vi "HFRR ADV v039.vi"() -> ()   [LabVIEW 2025] (continued)
                    n2649 = local read "Elapsed time"() -> (w3262:dbl)
                    n2650 = local read "AIR TEMP"() -> (w3235:dbl)
                    n2651 = local read "PID-out"() -> (w3240:dbl)
                    n2652 = local write "Temperature ( Deg C )"(w3231) -> ()
                    n2653 = Number To Fractional String(number=w3209, width (-)=i16 9 ("precision (6)"), precision (6)=i16 6) -> (F-format string=w3255:string)  [unwired: 1 in]
                    n2654 = Number To Fractional String(number=w3235, width (-)=i16 9 ("precision (6)"), precision (6)=i16 3) -> (F-format string=w3254:string)  [unwired: 1 in]
                    n2655 = Number To Fractional String(number=w3231, width (-)=i16 9 ("precision (6)"), precision (6)=i16 3) -> (F-format string=w3251:string)  [unwired: 1 in]
                    n2656 = Number To Fractional String(number=w3230, width (-)=i16 9 ("precision (6)"), precision (6)=i16 3) -> (F-format string=w3248:string)  [unwired: 1 in]
                    n2657 = Number To Fractional String(number=0.0, width (-)=i16 9 ("precision (6)"), precision (6)=i16 3) -> (F-format string=w3245:string)  [unwired: 1 in]
                    n2658 = Number To Fractional String(number=w3240, width (-)=i16 9 ("precision (6)"), precision (6)=i16 3) -> (F-format string=w3241:string)  [unwired: 1 in]
                    n2659 = Number To Fractional String(number=w3237, width (-)=i16 9 ("precision (6)"), precision (6)=i16 3) -> (F-format string=w3236:string)  [unwired: 1 in]
                    n2660 = Number To Fractional String(number=w3228, width (-)=i16 9 ("precision (6)"), precision (6)=i16 6) -> (F-format string=w3263:string)  [unwired: 1 in]
                    n2661 = Number To Fractional String(number=w3262, width (-)=i16 14 ("precision (6)"), precision (6)=i16 3) -> (F-format string=w3264:string)  [unwired: 1 in]
                    n2662 = Bundle("y"=1.02, "LVDT STROKE DISPLAY"=w3209, "y"=0.98) -> (w3229:T31)  [unwired: 1 in]
                    n2663 = Number To Fractional String(number="Ambient Humidity :", width (-)=i16 9 ("precision (6)"), precision (6)=i16 6) -> (F-format string=w3221:string)  [unwired: 1 in]
                    n2664 = local read "RUN"() -> (w3227:bool)
                    n2665 = case shown="True" w3227 {
                      tunnel: w3229 -> [_ w3280]
                      tunnel: w3209 -> [_ w3279]
                      tunnel: w3209 -> [_ w3277]
                      tunnel: w3209 -> [_ w3278]
                      frame False {
                      }
                      frame True {
                        "Stroke ( mm )" <- w3280
                        "Stroke ( mm )" <- w3280
                        "Stroke 4" <- w3279
                        "Stroke 3" <- w3277
                        "Stroke 2" <- w3278
                        "measured_stroke" <- w3277
                      }
                    }
                    n2666 = Concatenate Strings(w3264, w3223, w3263, w3223, w3255, w3223, w3254, w3223, w3251, w3223, w3248, w3223, w3245, w3223, w3241, w3223, w3236, w3223, w3221, "\r") -> (w3261:string)
                    n2667 = call <vilib>:"Write Characters To File.vi"("append to file? (new file:F)"=TRUE, "character string"=w3261, "file path (dialog if empty)"=w3214) -> ()  [unwired: 2 in, 1 out]
                    "refresh flag" <- TRUE ("refresh flag")
                    "LVDT STROKE Actual" <- w3207
                  }
                }
                n2668 = case shown="True" w3129 {
                  tunnel: w3139 -> [_ w3165]
                  tunnel: w3144 -> [_ w3175]
                  tunnel: [0.0 w3171] -> _
                  tunnel: w3138 -> [_ w3170]
                  tunnel: [0.0 w3169] -> _
                  tunnel: w3128 -> [_ w3169]
                  tunnel: w3142 -> [w3158 _]
                  frame False {
                    n2669 = local write "acq timer"(w3158) -> ()
                    n2670 = local write "Test Duration Status"(0.0 ("Test Duration Status")) -> ()
                  }
                  frame True {
                    n2671 = local read "Set Hz"() -> (w3172:dbl)
                    n2672 = local write "Elapsed time"(w3165) -> ()
                    n2673 = local read "test time"() -> (w3164:dbl)
                    n2674 = Multiply(x=w3175, y=w3172) -> (x*y=w3174:dbl)
                    n2675 = case shown="False" w3170 {
                      tunnel: w3174 -> [w3176 _]
                      tunnel: [w3176 1.0] -> w3171
                      frame False {
                        n2676 = local write "Cycles elapsed"(w3176) -> ()
                      }
                      frame True {
                      }
                    }
                    n2677 = Greater?(x=w3165, y=w3164) -> (0:w3173:bool)
                    n2678 = Subtract(x=w3164, y=w3165) -> (x-y=w3163:dbl)
                    n2679 = Multiply(x=w3163, y=60.0) -> (x*y=w3162:dbl)
                    n2680 = local write "Time Remaining"(w3162) -> ()
                    n2681 = local write "Remaining Time"(w3162) -> ()
                    n2682 = case shown="True" w3173 {
                      frame False {
                      }
                      frame True {
                        n2683 = stacked-sequence {
                          frame #0 {
                            w3181 = T19."Enabled" ("Disabled")
                            w3180 = FALSE ("TEST FILE NAM,E SAVED")
                            w3182 = "" ("FILE")
                            w3183 = TRUE ("Visible")
                            n2684 = local write "Humidity"(FALSE ("Humidity")) -> ()
                            n2685 = local write "RUN"(FALSE ("OK Button 2")) -> ()
                            n2686 = local write "Heater Button"(FALSE ("Heater Button")) -> ()
                            n2687 = local write "Auto Start Test"(FALSE ("Auto Start Test")) -> ()
                            n2688 = local write "TestCompFlg"(TRUE ("StpFlg")) -> ()
                            n2689 = local read "Humidity ( %RH )"() -> (→"Rh After":dbl)
                            n2690 = property on="STOP 2" class="Bool (strict)"("Disabled"=u8 0) -> ()  [unwired: 2 in, 2 out]
                            n2691 = local read "EVENT LOG"() -> (w3188:string)
                            n2692 = call "Event Log.vi"("Content"="Test Completed", "EVENT LOG"=w3188) -> ("EVENT LOG"=w3187:string)  [unwired: 8 in, 1 out]
                            n2693 = property on="RUN" class="Bool (strict)"("Visible"=w3183) -> ()  [unwired: 2 in, 2 out]
                            n2694 = property on="Auto Start Test" class="Bool (strict)"("Visible"=w3183) -> ()  [unwired: 2 in, 2 out]
                            n2695 = local write "Batch Ref Num :"(w3182) -> ()
                            n2696 = local write "FILE"(w3182) -> ()
                            n2697 = local write "EVENT LOG"(w3187) -> ()
                            n2698 = local write "TEST FILE NAM,E SAVED"(w3180) -> ()
                            n2699 = local write "Fuel Discription :"(w3182) -> ()
                            n2700 = local write "START TEMP"(w3180) -> ()
                            n2701 = local write "Remarks :"(w3182) -> ()
                            n2702 = local write "Main Dashboard Buttons"(T1."Imaging" ("Main Dashboard Buttons")) -> ()
                            n2703 = local write "Main Tab"(T2."Adv Scar" ("Main Tab")) -> ()
                            n2704 = property on="FRICVALZ 2" class="Bool (strict)"("DisabledEnum"=w3181) -> ()  [unwired: 2 in, 2 out]
                            n2705 = property on="FRICVALZ 3" class="Bool (strict)"("DisabledEnum"=w3181) -> ()  [unwired: 2 in, 2 out]
                            n2706 = property on="FRICVALZ 4" class="Bool (strict)"("DisabledEnum"=w3181) -> ()  [unwired: 2 in, 2 out]
                          }
                          frame #1 {
                            n2707 = Wait (ms)(milliseconds to wait=u32 1500) -> ()  [unwired: 1 out]
                          }
                          frame #2 {
                            n2708 = local write "Due Write"("VC;0") -> ()
                          }
                          frame #3 {
                            n2709 = Wait (ms)(milliseconds to wait=u32 1500) -> ()  [unwired: 1 out]
                          }
                          frame #4 {
                            n2710 = local write "Due Write"("VC;0") -> ()
                          }
                          frame #5 {
                            n2711 = Wait (ms)(milliseconds to wait=u32 1500) -> ()  [unwired: 1 out]
                          }
                          frame #6 {
                            n2712 = local write "Due Write"("ST;0") -> ()
                          }
                          frame #7 {
                            n2713 = local write "measured_stroke"(0.0 ("measured_stroke")) -> ()
                            n2714 = Wait (ms)(milliseconds to wait=u32 1500) -> ()  [unwired: 1 out]
                          }
                          frame #8 {
                            n2715 = local write "Due Write"("HE;0") -> ()
                            n2716 = local write "Humidity 2"(TRUE ("Humidity")) -> ()
                          }
                        }
                      }
                    }
                    n2717 = Divide(x=w3165, y=w3164) -> (x/y=w3168:dbl)
                    n2718 = Multiply(x=w3168, y=100.0) -> (x*y=w3166:dbl)
                    n2719 = local write "Test Duration Status"(w3166) -> ()
                  }
                }
              }
              frame #2 {
                n2720 = case shown="True" "Heater Button" {
                  tunnel: [0.0 ("output") w3303] -> w3281
                  frame False {
                    w3284 = TRUE ("tmpchk")
                    n2721 = local read "TEMP"() -> (w3285:dbl)
                    n2722 = local write "Temp ini"(w3285) -> ()
                    n2723 = local write "Reset 4"(w3284) -> ()
                    n2724 = local write "tmpchk"(w3284) -> ()
                    n2725 = local write "reinit"(TRUE ("reinit")) -> ()
                    n2726 = local write "manual temp log"(TRUE ("manual temp log")) -> ()
                  }
                  frame True {
                    # "Logic to turn off\nthe heater when \ntemp is not rising.\nTime - 60 sec\nDelta t- 5°c"
                    n2727 = local read "Temp ini"() -> (w3292:dbl)
                    n2728 = local read "Auto Start Test"() -> (w3288:bool)
                    n2729 = Less?(x=w3292, y=53.0) -> (x < y?=w3290:bool)
                    n2730 = case shown="False" w3288 {
                      frame False {
                        n2731 = local read "Set Temp"() -> (w3312:dbl)
                        n2732 = local read "TEMP"() -> (w3311:dbl)
                        n2733 = Subtract(x=w3312, y=w3311) -> (x-y=w3310:dbl)
                        n2734 = Absolute Value(x=w3310) -> (abs(x)=w3309:dbl)
                        n2735 = Less?(x=w3309, y=0.5) -> (x < y?=w3307:bool)
                        n2736 = case shown="True" w3307 {
                          tunnel: "manual temp log" -> [_ w3313]
                          frame False {
                          }
                          frame True {
                            n2737 = case shown="True" w3313 {
                              selector: w3313 -> [_ w3314]
                              frame False {
                              }
                              frame True {
                                # "#Event log"
                                n2738 = Not(x=w3314) -> (.not. x?=w3315:bool)
                                n2739 = local write "manual temp log"(w3315) -> ()
                                n2740 = local read "EVENT LOG"() -> (w3318:string)
                                n2741 = call "Event Log.vi"("Content"="Target Temperature reached", "EVENT LOG"=w3318) -> ("EVENT LOG"=w3317:string)  [unwired: 8 in, 1 out]
                                n2742 = local write "EVENT LOG"(w3317) -> ()
                              }
                            }
                          }
                        }
                      }
                      frame True {
                        n2743 = local write "manual temp log"(TRUE ("manual temp log")) -> ()
                      }
                    }
                    n2744 = And(x="tmpchk", y=w3290) -> (x .and. y?=w3293:bool)
                    n2745 = case shown="True" w3293 {
                      frame False {
                      }
                      frame True {
                        n2746 = call "Elapsed Time8"("Time Target (s)"=300.0, "Reset"="Reset 4") -> ("Time has Elapsed"=w3320:bool)  [unwired: 10 in, 7 out]
                        n2747 = flat-sequence {
                          tunnel: w3320 -> [_]
                          frame #0 {
                            n2748 = local write "Reset 4"(FALSE ("Reset 4")) -> ()
                          }
                        }
                        n2749 = case shown="True" w3320 {
                          frame False {
                          }
                          frame True {
                            n2750 = local read "Temp ini"() -> (w3327:dbl)
                            n2751 = Add(x=w3327, y=5.0) -> (x+y=w3325:dbl)
                            n2752 = local read "TEMP"() -> (w3328:dbl)
                            n2753 = Greater?(x=w3328, y=w3325) -> (0:w3326:bool)
                            n2754 = case shown="False" w3326 {
                              frame False {
                                n2755 = local write "Heater Button"(FALSE ("Heater Button")) -> ()
                              }
                              frame True {
                                n2756 = local write "tmpchk"(FALSE ("tmpchk")) -> ()
                              }
                            }
                          }
                        }
                      }
                    }
                    n2757 = local read "Set Temp"() -> (w3301:dbl)
                    n2758 = local read "TEMP"() -> (w3295:dbl)
                    n2759 = call-poly <vilib>:"PID.vi"("reinitialize? (F)"="reinit", "dt (s)"=-1.0, "process variable"=w3295, "setpoint"=w3301) -> ("output"=w3298:dbl)  [unwired: 6 in, 1 out]
                    n2760 = Subtract(x=w3301, y=w3295) -> (x-y=w3302:dbl)
                    n2761 = Add(x=w3301, y=0.5) -> (x+y=w3299:dbl)
                    n2762 = Greater Or Equal?(x=w3295, y=w3299) -> ()  [unwired: 1 out]
                    n2763 = Select(t=0.0, s=FALSE, f=w3298) -> (s? t:f=w3297:dbl)
                    "PID output" <- w3297
                    n2764 = flat-sequence {
                      tunnel: w3297 -> [w3331]
                      tunnel: [w3331] -> w3303
                      frame #0 {
                        n2765 = local write "reinit"(FALSE ("reinit")) -> ()
                      }
                    }
                    n2766 = Bundle(w3302, "output"=w3297, "TEMP"=w3295) -> ()  [unwired: 1 in, 1 out]
                  }
                }
                "PID-out" <- w3281
              }
              frame #3 {
                n2767 = local read "TEMP"() -> (w3333:dbl)
                n2768 = Greater Or Equal?(x=w3333, y="Set Temp 2") -> (x >= y?=w3338:bool)
                n2769 = case shown="True" w3338 {
                  tunnel: [FALSE TRUE] -> w3336
                  frame False {
                  }
                  frame True {
                  }
                }
                "Status 13" <- w3336
                n2770 = And(x=w3336, y="trip1 8") -> (x .and. y?=w3335:bool)
                n2771 = case shown="True" w3335 {
                  frame False {
                    n2772 = local write "Heater Trip Temp"(TRUE ("Heater Trip Temp")) -> ()
                  }
                  frame True {
                    w3341 = FALSE ("OK Button 2")
                    n2773 = case shown="True" "Heater Trip Temp" {
                      selector: "Heater Trip Temp" -> [_ w3343]
                      frame False {
                      }
                      frame True {
                        n2774 = Not(x=w3343) -> (.not. x?=w3342:bool)
                        n2775 = local read "EVENT LOG"() -> (w3346:string)
                        n2776 = local write "Heater Trip Temp"(w3342) -> ()
                        n2777 = call "Event Log.vi"("Content"="Heater Trip", "EVENT LOG"=w3346) -> ("EVENT LOG"=w3345:string)  [unwired: 8 in, 1 out]
                        n2778 = local write "EVENT LOG"(w3345) -> ()
                      }
                    }
                    n2779 = local write "RUN"(w3341) -> ()
                    n2780 = property on="Auto Start Test" class="Bool (strict)"("Value"=w3341) -> ()  [unwired: 2 in, 2 out]
                    n2781 = local write "Heater Button"(w3341) -> ()
                  }
                }
              }
            }
            n2782 = case shown="False" w3052 {
              frame False {
                n2783 = disable-structure shown="Disabled" {
                  frame Disabled {
                    n2784 = stacked-sequence {
                      frame #0 {
                        n2785 = local write "RUN"(FALSE ("OK Button 2")) -> ()
                      }
                      frame #1 {
                      }
                    }
                  }
                  frame Enabled {
                  }
                }
              }
              frame True {
              }
            }
          }
        }
        n2786 = local read "Reset Graph"() -> (w2949:bool)
        n2787 = case shown="True" w2949 {
          selector: w2949 -> [_ w2966]
          frame False {
          }
          frame True {
            w2980 = 0.0 ("X Scale.Range:Maximum")
            n2788 = Not(x=w2966) -> (.not. x?=w2965:bool)
            n2789 = local write "Reset Graph"(w2965) -> ()
            n2790 = property on="Electrical Contact Resistance ( % )" class="WFChart (strict)"("XScale.Maximum"=600.0 ("X Scale.Range:Maximum"), "XScale.Minimum"=0.0 ("X Scale.Range:Minimum"), "YScale.Maximum"=100.0 ("Y Scale.Range:Maximum"), "YScale.Minimum"=0.0 ("Y Scale.Range:Minimum")) -> ()  [unwired: 2 in, 2 out]
            n2791 = property on="Frictional Force ( N )" class="WFChart (strict)"("XScale.Maximum"=600.0 ("X Scale.Range:Maximum"), "XScale.Minimum"=0.0 ("X Scale.Range:Minimum"), "YScale.Maximum"=100.0 ("Y Scale.Range:Maximum"), "YScale.Minimum"=0.0 ("Y Scale.Range:Minimum")) -> ()  [unwired: 2 in, 2 out]
            n2792 = property on="Temperature ( Deg C )" class="WFChart (strict)"("XScale.Maximum"=600.0 ("X Scale.Range:Maximum"), "XScale.Minimum"=0.0 ("X Scale.Range:Minimum"), "YScale.Maximum"=100.0 ("Y Scale.Range:Maximum"), "YScale.Minimum"=0.0 ("Y Scale.Range:Minimum")) -> ()  [unwired: 2 in, 2 out]
            n2793 = property on="Stroke ( mm )" class="WFChart (strict)"("XScale.Maximum"=600.0 ("X Scale.Range:Maximum"), "XScale.Minimum"=0.0 ("X Scale.Range:Minimum"), "YScale.Maximum"=100.0 ("Y Scale.Range:Maximum"), "YScale.Minimum"=0.0 ("Y Scale.Range:Minimum")) -> ()  [unwired: 2 in, 2 out]
            n2794 = property on="Coefficient of Friction" class="WFChart (strict)"("XScale.Maximum"=600.0 ("X Scale.Range:Maximum"), "XScale.Minimum"=0.0 ("X Scale.Range:Minimum"), "YScale.Maximum"=100.0 ("Y Scale.Range:Maximum"), "YScale.Minimum"=0.0 ("Y Scale.Range:Minimum")) -> ()  [unwired: 2 in, 2 out]
            n2795 = property on="Electrical Contact Resistance ( % )" class="WFChart (strict)"("XScale.Minimum"=0.0 ("X Scale.Range:Minimum"), "XScale.Maximum"=600.0 ("X Scale.Range:Maximum"), "YScale.Minimum"=0.0 ("Y Scale.Range:Minimum"), "YScale.Maximum"=100.0 ("Y Scale.Range:Maximum")) -> ()  [unwired: 2 in, 2 out]
            n2796 = property on="Temperature ( Deg C )" class="WFChart (strict)"("XScale.Minimum"=0.0 ("X Scale.Range:Minimum"), "XScale.Maximum"=600.0 ("X Scale.Range:Maximum"), "YScale.Minimum"=0.0 ("Y Scale.Range:Minimum"), "YScale.Maximum"=100.0 ("Y Scale.Range:Maximum")) -> ()  [unwired: 2 in, 2 out]
            n2797 = property on="Coefficient of Friction" class="WFChart (strict)"("XScale.Minimum"=0.0 ("X Scale.Range:Minimum"), "XScale.Maximum"=600.0 ("X Scale.Range:Maximum"), "YScale.Maximum"=1.0 ("X Scale.Range:Minimum"), "YScale.Minimum"=0.0 ("X Scale.Range:Minimum")) -> ()  [unwired: 2 in, 2 out]
            n2798 = property on="Frictional Force ( N )" class="WFChart (strict)"("XScale.Maximum"=600.0 ("X Scale.Range:Maximum"), "XScale.Minimum"=w2980, "YScale.Maximum"=10.0 ("Y Scale.Range:Maximum"), "YScale.Minimum"=w2980) -> ()  [unwired: 2 in, 2 out]
            n2799 = property on="Stroke ( mm )" class="WFChart (strict)"("XScale.Maximum"=600.0 ("X Scale.Range:Maximum"), "XScale.Minimum"=0.0 ("X Scale.Range:Minimum"), "YScale.Maximum"=100.0 ("Y Scale.Range:Maximum"), "YScale.Minimum"=0.0 ("Y Scale.Range:Minimum")) -> ()  [unwired: 2 in, 2 out]
          }
        }
      }
      frame "Compare Files" {
        # "Elapsed time\ncof\nstroke\nAir temp\nTemp\nHumidity"
        n2800 = case shown="True" "RSTV1 2" {
          frame False {
          }
          frame True {
            n2801 = property on="Humidity ( %RH )" class="XYGraph (strict)"("Y Scale.Display Format:Precision"=u8 0 ("Y Scale.Format & Precision:Precision")) -> ()  [unwired: 2 in, 2 out]
            n2802 = property on="Humidity ( %RH )" class="XYGraph (strict)"("X Scale.Range:Minimum"=0.0, "X Scale.Range:Maximum"=75.0, "Y Scale.Range:Minimum"=48.0, "Y Scale.Range:Maximum"=58.0) -> ()  [unwired: 2 in, 2 out]
          }
        }
        n2803 = case shown="True" "RST CP 2" {
          frame False {
          }
          frame True {
            n2804 = property on="XY Graph 13" class="XYGraph (strict)"("Y Scale.Display Format:Precision"=u8 0 ("Y Scale.Format & Precision:Precision")) -> ()  [unwired: 2 in, 2 out]
            n2805 = property on="XY Graph 13" class="XYGraph (strict)"("X Scale.Range:Minimum"=0.0, "X Scale.Range:Maximum"=75.0, "Y Scale.Range:Minimum"=0.0, "Y Scale.Range:Maximum"=100.0) -> ()  [unwired: 2 in, 2 out]
          }
        }
        n2806 = case shown="True" "RST CP" {
          frame False {
          }
          frame True {
            n2807 = property on="Sample Temperature ( °C )" class="XYGraph (strict)"("Y Scale.Display Format:Precision"=u8 2 ("Y Scale.Format & Precision:Precision")) -> ()  [unwired: 2 in, 2 out]
            n2808 = property on="Sample Temperature ( °C )" class="XYGraph (strict)"("X Scale.Range:Minimum"=0.0, "X Scale.Range:Maximum"=75.0, "Y Scale.Range:Minimum"=58.0, "Y Scale.Range:Maximum"=62.0) -> ()  [unwired: 2 in, 2 out]
          }
        }
        n2809 = case shown="True" "RSTV1 3" {
          frame False {
          }
          frame True {
            n2810 = property on="Air Temperature  ( °C )" class="XYGraph (strict)"("Y Scale.Display Format:Precision"=u8 2 ("Y Scale.Format & Precision:Precision")) -> ()  [unwired: 2 in, 2 out]
            n2811 = property on="Air Temperature  ( °C )" class="XYGraph (strict)"("X Scale.Range:Minimum"=0.0 ("Y Scale.Range:Minimum"), "X Scale.Range:Maximum"=75.0 ("Y Scale.Range:Maximum"), "Y Scale.Range:Minimum"=20.0 ("X Scale.Range:Minimum"), "Y Scale.Range:Maximum"=26.0 ("X Scale.Range:Maximum")) -> ()  [unwired: 2 in, 2 out]
          }
        }
        n2812 = case shown="True" "RSTV1 4" {
          frame False {
          }
          frame True {
            n2813 = property on="Stroke ( mm )" class="XYGraph (strict)"("Y Scale.Display Format:Precision"=u8 2 ("Y Scale.Format & Precision:Precision")) -> ()  [unwired: 2 in, 2 out]
            n2814 = property on="Stroke ( mm )" class="XYGraph (strict)"("X Scale.Range:Minimum"=0.0 ("Y Scale.Range:Maximum"), "X Scale.Range:Maximum"=75.0 ("X Scale.Range:Minimum"), "Y Scale.Range:Minimum"=0.98, "Y Scale.Range:Maximum"=1.02) -> ()  [unwired: 2 in, 2 out]
          }
        }
        n2815 = case shown="True" "rstv2" {
          frame False {
          }
          frame True {
            n2816 = property on="Coefficient Of Friction" class="XYGraph (strict)"("Y Scale.Display Format:Precision"=u8 3 ("Y Scale.Format & Precision:Precision")) -> ()  [unwired: 2 in, 2 out]
            n2817 = property on="Coefficient Of Friction" class="XYGraph (strict)"("X Scale.Range:Minimum"=0.0 ("Y Scale.Range:Maximum"), "X Scale.Range:Maximum"=75.0, "Y Scale.Range:Minimum"=0.0, "Y Scale.Range:Maximum"=1.0 ("X Scale.Range:Minimum")) -> ()  [unwired: 2 in, 2 out]
          }
        }
        n2818 = case shown="True" "RST CP 3" {
          frame False {
          }
          frame True {
            n2819 = property on="Air Temp ( °C ) vs Humidity ( % RH )" class="XYGraph (strict)"("X Scale.Range:Minimum"=18.0, "X Scale.Range:Maximum"=28.0 ("X Scale.Range:Minimum"), "Y Scale.Range:Minimum"=30.0 ("X Scale.Range:Minimum"), "Y Scale.Range:Maximum"=70.0 ("X Scale.Range:Minimum")) -> ()  [unwired: 2 in, 2 out]
          }
        }
        n2820 = case shown="True" "OPEN 1" {
          frame False {
          }
          frame True {
            (unwired) 0  # existing file
            w3622 = "Choose a datalog file to open"  # prompt
            n2821 = local write "OPEN 1"(FALSE ("OPEN 1")) -> ()
            n2822 = String To Path(string="C:\\LAB-IQ\\Data\\") -> (path=w3607:path)
            n2823 = File Dialog(6:"*.dgf" ("pattern"), 7:w3622, 11:w3607) -> (0:w3605:errorcluster, 3:w3613:path)  [unwired: 4 in, 2 out]
            n2824 = Unbundle(w3605) -> ()  [unwired: 3 out]
            n2825 = Strip Path(path=w3613) -> (name=w3612:string)  [unwired: 1 out]
            n2826 = Path To String(path=w3613) -> (string=w3608:string)
            "string1" <- w3608
            n2827 = Match Pattern(string=w3612, regular expression=".dgf") -> (before substring=→"String Control":string)  [unwired: 1 in, 3 out]
            n2828 = Match Pattern(string=w3608, regular expression=".dgf" ("substring (\"\")")) -> (before substring=w3618:string)  [unwired: 1 in, 3 out]
            n2829 = Concatenate Strings(w3618, ".duf" ("Substring")) -> (w3614:string)
            n2830 = String To Path(string=w3614) -> (path=w3619:path)
            n2831 = call <vilib>:"Read Characters From File.vi"("file path (dialog if empty)"=w3619, "start of read offset (chars.:0)"=60 ("start of read offset (chars.: 0)")) -> ("character string"=→"String Control 2":string)  [unwired: 4 in, 3 out]
          }
        }
        n2832 = case shown="True" "OPEN 2" {
          frame False {
          }
          frame True {
            (unwired) 0  # existing file
            w3640 = "Choose a datalog file to open"  # prompt
            n2833 = local write "OPEN 2"(FALSE ("OPEN 1")) -> ()
            n2834 = String To Path(string="C:\\LAB-IQ\\Data\\") -> (path=w3625:path)
            n2835 = File Dialog(6:"*.dgf" ("pattern"), 7:w3640, 11:w3625) -> (0:w3623:errorcluster, 3:w3631:path)  [unwired: 4 in, 2 out]
            n2836 = Unbundle(w3623) -> ()  [unwired: 3 out]
            n2837 = Strip Path(path=w3631) -> (name=w3629:string)  [unwired: 1 out]
            n2838 = Path To String(path=w3631) -> (string=w3626:string)
            "string1 2" <- w3626
            n2839 = Match Pattern(string=w3629, regular expression=".dgf") -> (before substring=→"String Control 3":string)  [unwired: 1 in, 3 out]
            n2840 = Match Pattern(string=w3626, regular expression=".dgf" ("substring (\"\")")) -> (before substring=w3637:string)  [unwired: 1 in, 3 out]
            n2841 = Concatenate Strings(w3637, ".duf" ("Substring")) -> (w3634:string)
            n2842 = String To Path(string=w3634) -> (path=w3632:path)
            n2843 = call <vilib>:"Read Characters From File.vi"("file path (dialog if empty)"=w3632, "start of read offset (chars.:0)"=60 ("start of read offset (chars.: 0)")) -> ("character string"=→"String Control 4":string)  [unwired: 4 in, 3 out]
          }
        }
        n2844 = case shown="True" "OPEN 3" {
          frame False {
          }
          frame True {
            (unwired) 0  # existing file
            w3658 = "Choose a datalog file to open"  # prompt
            n2845 = local write "OPEN 3"(FALSE ("OPEN 1")) -> ()
            n2846 = String To Path(string="C:\\LAB-IQ\\Data\\") -> (path=w3643:path)
            n2847 = File Dialog(6:"*.dgf" ("pattern"), 7:w3658, 11:w3643) -> (0:w3641:errorcluster, 3:w3649:path)  [unwired: 4 in, 2 out]
            n2848 = Unbundle(w3641) -> ()  [unwired: 3 out]
            n2849 = Strip Path(path=w3649) -> (name=w3647:string)  [unwired: 1 out]
            n2850 = Path To String(path=w3649) -> (string=w3644:string)
            "string1 3" <- w3644
            n2851 = Match Pattern(string=w3647, regular expression=".dgf") -> (before substring=→"String Control 5":string)  [unwired: 1 in, 3 out]
            n2852 = Match Pattern(string=w3644, regular expression=".dgf" ("substring (\"\")")) -> (before substring=w3654:string)  [unwired: 1 in, 3 out]
            n2853 = Concatenate Strings(w3654, ".duf" ("Substring")) -> (w3651:string)
            n2854 = String To Path(string=w3651) -> (path=w3655:path)
            n2855 = call <vilib>:"Read Characters From File.vi"("file path (dialog if empty)"=w3655, "start of read offset (chars.:0)"=60 ("start of read offset (chars.: 0)")) -> ("character string"=→"String Control 6":string)  [unwired: 4 in, 3 out]
          }
        }
        n2856 = case shown="True" "OPEN 4" {
          frame False {
          }
          frame True {
            (unwired) 0  # existing file
            w3676 = "Choose a datalog file to open"  # prompt
            n2857 = local write "OPEN 4"(FALSE ("OPEN 1")) -> ()
            n2858 = String To Path(string="C:\\LAB-IQ\\Data\\") -> (path=w3661:path)
            n2859 = File Dialog(6:"*.dgf" ("pattern"), 7:w3676, 11:w3661) -> (0:w3659:errorcluster, 3:w3667:path)  [unwired: 4 in, 2 out]
            n2860 = Unbundle(w3659) -> ()  [unwired: 3 out]
            n2861 = Strip Path(path=w3667) -> (name=w3665:string)  [unwired: 1 out]
            n2862 = Path To String(path=w3667) -> (string=w3662:string)
            "string1 4" <- w3662
            n2863 = Match Pattern(string=w3665, regular expression=".dgf") -> (before substring=→"String Control 7":string)  [unwired: 1 in, 3 out]
            n2864 = Match Pattern(string=w3662, regular expression=".dgf" ("substring (\"\")")) -> (before substring=w3672:string)  [unwired: 1 in, 3 out]
            n2865 = Concatenate Strings(w3672, ".duf" ("Substring")) -> (w3669:string)
            n2866 = String To Path(string=w3669) -> (path=w3673:path)
            n2867 = call <vilib>:"Read Characters From File.vi"("file path (dialog if empty)"=w3673, "start of read offset (chars.:0)"=60 ("start of read offset (chars.: 0)")) -> ("character string"=→"String Control 8":string)  [unwired: 4 in, 3 out]
          }
        }
      }
      frame "About" {
        # "Elapsed time\ncof\nstroke\nmean pos\nTemp\nHumidity"
        n2868 = disable-structure shown="Disabled" {
          frame Disabled {
            n2869 = case shown="True" "Export" {
              frame False {
              }
              frame True {
                w3698 = "                                      " ("string")
                w3700 = "\r"
                (unwired) i16 6 ("width (-)")
                w3777 = "\r"
                w3709 = "\r"
                n2870 = local write "Export"(FALSE ("Export")) -> ()
                n2871 = local read "String 29"() -> (w3746:string)
                n2872 = local read "String 34"() -> (w3734:string)
                n2873 = local read "String 35"() -> (w3729:string)
                n2874 = local read "String 37"() -> (w3725:string)
                n2875 = local read "String 36"() -> (w3722:string)
                n2876 = local read "String 38"() -> (w3719:string)
                n2877 = local read "String 39"() -> (w3716:string)
                n2878 = Match Pattern(string=w3746, regular expression=".dwm") -> (before substring=w3742:string)  [unwired: 1 in, 3 out]
                "before substring" <- w3742
                n2879 = local read "S 38"() -> (w3737:string)
                n2880 = local read "S 39"() -> (w3730:string)
                n2881 = local read "Temperature before test 2"() -> (w3766:dbl)
                n2882 = local read "Temperature after test 2"() -> (w3771:dbl)
                n2883 = local read "Humidity before test 2"() -> (w3752:dbl)
                n2884 = local read "Humidity after test 2"() -> (w3767:dbl)
                n2885 = local read "MWSD 2"() -> (w3763:dbl)
                n2886 = local read "WS1.4 2"() -> (w3779:dbl)
                n2887 = local read "HCF 2"() -> (w3775:dbl)
                n2888 = local read "AVP 2"() -> (w3764:dbl)
                n2889 = Concatenate Strings("1," ("string"), w3737) -> (w3736:string)
                n2890 = Concatenate Strings("2," ("string"), w3734) -> (w3733:string)
                n2891 = Concatenate Strings("3," ("string"), w3730) -> (w3732:string)
                n2892 = Concatenate Strings("4," ("string"), w3729) -> (w3728:string)
                n2893 = Concatenate Strings("5," ("string"), w3725) -> (w3726:string)
                n2894 = Concatenate Strings("6," ("string"), w3722) -> (w3723:string)
                n2895 = Concatenate Strings("7," ("string"), w3719) -> (w3720:string)
                n2896 = Concatenate Strings("8," ("string"), w3716) -> (w3717:string)
                n2897 = local read "Sample ID"() -> (w3784:string)
                n2898 = case shown="\"xlx\"" "Select File Type" {
                  tunnel: w3742 -> [w3787 w3789 w3791]
                  tunnel: [w3785 w3790 w3792] -> w3741
                  frame "xlx" {
                    n2899 = Concatenate Strings(w3787, ".xls" ("string")) -> (w3785:string)
                  }
                  frame "csv" {
                    n2900 = Concatenate Strings(w3789, ".csv" ("string")) -> (w3790:string)
                  }
                  frame "txt" {
                    n2901 = Concatenate Strings(w3791, ".txt" ("string")) -> (w3792:string)
                  }
                }
                n2902 = local read "Test Date"() -> (w3783:string)
                n2903 = local read "String 45"() -> (w3697:string)
                n2904 = local read "String 31"() -> (w3782:string)
                n2905 = local read "String 32"() -> (w3781:string)
                n2906 = local read "TITTLE"() -> (w3705:string)
                n2907 = Number To Fractional String(number=w3752, width (-)=i16 6, precision (6)=i16 2) -> (F-format string=w3751:string)  [unwired: 1 in]
                n2908 = Number To Fractional String(number=w3766, width (-)=i16 6, precision (6)=i16 2) -> (F-format string=w3772:string)  [unwired: 1 in]
                n2909 = Number To Fractional String(number=w3767, width (-)=i16 6, precision (6)=i16 2) -> (F-format string=w3765:string)  [unwired: 1 in]
                n2910 = Number To Fractional String(number=w3771, width (-)=i16 6, precision (6)=i16 2) -> (F-format string=w3770:string)  [unwired: 1 in]
                n2911 = Number To Fractional String(number=w3763, width (-)=i16 6, precision (6)=i16 2) -> (F-format string=w3761:string)  [unwired: 1 in]
                n2912 = Number To Fractional String(number=w3764, width (-)=i16 6, precision (6)=i16 2) -> (F-format string=w3762:string)  [unwired: 1 in]
                n2913 = Number To Fractional String(number=w3775, width (-)=i16 6, precision (6)=i16 2) -> (F-format string=w3776:string)  [unwired: 1 in]
                n2914 = Number To Fractional String(number=w3779, precision (6)=i16 2) -> (F-format string=w3780:string)  [unwired: 2 in]
                n2915 = local read "s.NO"() -> (w3699:string)
                n2916 = Concatenate Strings("=" ("string"), w3705) -> (w3704:string)
                n2917 = Concatenate Strings("S.No," ("string"), "                                       Parameters" ("string")) -> (w3710:string)
                n2918 = Concatenate Strings(w3777, w3736, w3751, w3777, w3733, w3772, w3777, w3732, w3765, w3777, w3728, w3770, w3777, w3726, w3761, w3777, w3723, w3762, w3777, w3720, w3776, w3777, w3717, w3780) -> (w3739:string)
                n2919 = Concatenate Strings(w3709, "," ("string"), w3697, w3699, w3698, w3781, w3784, w3698, w3782, w3783, w3709) -> (w3707:string)
                n2920 = local read "Tested by"() -> (w3713:string)
                n2921 = local read "String 33"() -> (w3714:string)
                n2922 = Concatenate Strings("," ("string"), "                                                                             " ("string")) -> (w3702:string)
                n2923 = Concatenate Strings(w3704, w3700, w3707, w3700, w3710, w3739, w3700, w3702, w3714, w3713) -> (→"export":string)
                n2924 = String To Path(string=w3741) -> (path=w3748:path)
                n2925 = local read "export"() -> (w3743:string)
                n2926 = call <vilib>:"Write Characters To File.vi"("append to file? (new file:F)"=FALSE, "character string"=w3743, "file path (dialog if empty)"=w3748) -> ()  [unwired: 2 in, 1 out]
              }
            }
          }
          frame Enabled {
          }
        }
        n2927 = case shown="True" "OK Button 17" {
          frame False {
          }
          frame True {
            (unwired) 0  # existing file
            w4001 = "Choose a datalog file to open"  # prompt
            n2928 = local write "OK Button 17"(FALSE ("OK Button 17")) -> ()
            n2929 = local read "String"() -> (w3996:string)
            n2930 = String To Path(string=w3996) -> (path=w3997:path)
            n2931 = File Dialog(6:"*.duf" ("pattern"), 7:w4001, 11:w3997) -> (0:w3988:errorcluster, 3:w4007:path)  [unwired: 4 in, 2 out]
            n2932 = Unbundle(w3988) -> ()  [unwired: 3 out]
            n2933 = Open/Create/Replace File "Open File"(file path (use dialog)=w4007) -> (refnum out=w3999:refnum<file>)  [unwired: 5 in, 2 out]
            n2934 = Strip Path(path=w4007) -> (name=w4005:string)  [unwired: 1 out]
            n2935 = Path To String(path=w4007) -> (string=w3990:string)
            n2936 = while {
              tunnel: w3999 -> [w4011]
              i -> [w4008]
              stop <- w4009 continue-if-true
              (unwired) TRUE ("line mode (F)")
              n2937 = Read from Text File "Read File"(file (use dialog)=w4011) -> (text=w4010:string)  [unwired: 3 in, 3 out]
              n2938 = local write "Numeric 16"(w4008) -> ()
              n2939 = String Length(string=w4010) -> (length=w4013:i32)
              n2940 = Greater?(x=w4013, y=1) -> (0:w4009:bool)
            }
            n2941 = local write "String 29"(w3990) -> ()
            n2942 = Search and Replace String(input string=w3990, search string=".duf", replace string=".dgf" ("replace string (\"\")")) -> (result string=→"String Indicator 4":string)  [unwired: 5 in, 3 out]
            n2943 = Match Pattern(string=w4005, regular expression=".dwm") -> (before substring=w3989:string)  [unwired: 1 in, 3 out]
            "String Indicator" <- w3989
            n2944 = Match Pattern(string=w3990, regular expression=".dwm" ("substring (\"\")")) -> (before substring=w3991:string)  [unwired: 1 in, 3 out]
            "String Indicator 3" <- w3991
            n2945 = local write "TITTLE 2"(w3989) -> ()
            n2946 = String To Path(string=w3991) -> (path=w3998:path)
            "path" <- w3998
            n2947 = call <vilib>:"Read Characters From File.vi"("file path (dialog if empty)"=w3998, "start of read offset (chars.:0)"=60 ("start of read offset (chars.: 0)")) -> ("character string"=→"String Indicator 2":string)  [unwired: 4 in, 3 out]
          }
        }
        n2948 = call <vilib>:"Query Available Printers.vi"() -> ("system configured printers"=w3690:string[])  [unwired: 9 in, 2 out]
        "System Configured Printers 2" <- w3690
        n2949 = local read "OK Button 16"() -> (w3687:bool)
        n2950 = case shown="True" "OK Button 16" {
          frame False {
          }
          frame True {
            n2951 = stacked-sequence {
              frame #0 {
                n2952 = local read "Numeric 16"() -> (w4015:i32)
                n2953 = local write "Numeric 10"(w4015) -> ()
              }
              frame #1 {
                n2954 = local read "String 29"() -> (w4018:string)
                n2955 = String To Path(string=w4018) -> (path=w4017:path)
                n2956 = Open/Create/Replace File "Open File"(file path (use dialog)=w4017) -> (refnum out=w4019:refnum<file>)  [unwired: 5 in, 2 out]
                n2957 = for {
                  N: 16 -> [_]
                  tunnel: w4019 -> [w4026]
                  i -> [w4022]
                  (unwired) TRUE ("line mode (F)")
                  n2958 = Read from Text File "Read File"(file (use dialog)=w4026) -> (text=w4020:string)  [unwired: 3 in, 3 out]
                  n2959 = Match Pattern(string=w4020, regular expression="(") -> (after substring=w4025:string)  [unwired: 1 in, 3 out]
                  n2960 = Match Pattern(string=w4025, regular expression=")") -> (before substring=w4021:string)  [unwired: 1 in, 3 out]
                  n2961 = case shown="1" w4022 {
                    tunnel: w4021 -> [w4027 w4028 _ _ w4029 w4030 w4031 w4033 w4035 w4037 w4039 w4041 w4043 w4045 _]
                    tunnel: w4020 -> [_ _ _ _ _ _ _ _ _ _ _ _ _ _ _]
                    frame 0 {
                      "TITTLE" <- w4027
                    }
                    frame 1 {
                      "Sample ID" <- w4028
                    }
                    frame 2 {
                    }
                    frame 3 {
                    }
                    frame 4 {
                      "Test Date" <- w4029
                    }
                    frame 5 {
                      "Tested by" <- w4030
                    }
                    frame 6 {
                      n2962 = Fract/Exp String To Number(string=w4031) -> (number=→"Humidity before test 2":dbl)  [unwired: 3 in, 1 out]
                    }
                    frame 7 {
                      n2963 = Fract/Exp String To Number(string=w4033) -> (number=→"Temperature before test 2":dbl)  [unwired: 3 in, 1 out]
                    }
                    frame 8 {
                      n2964 = Fract/Exp String To Number(string=w4035) -> (number=→"Humidity after test 2":dbl)  [unwired: 3 in, 1 out]
                    }
                    frame 9 {
                      n2965 = Fract/Exp String To Number(string=w4037) -> (number=→"Temperature after test 2":dbl)  [unwired: 3 in, 1 out]
                    }
                    frame 10 {
                      n2966 = Fract/Exp String To Number(string=w4039) -> (number=→"MWSD 2":dbl)  [unwired: 3 in, 1 out]
                    }
                    frame 11 {
                      n2967 = Fract/Exp String To Number(string=w4041) -> (number=→"AVP 2":dbl)  [unwired: 3 in, 1 out]
                    }
                    frame 12 {
                      n2968 = Fract/Exp String To Number(string=w4043) -> (number=→"HCF 2":dbl)  [unwired: 3 in, 1 out]
                    }
                    frame 13 {
                      n2969 = Fract/Exp String To Number(string=w4045) -> (number=→"WS1.4 2":dbl)  [unwired: 3 in, 1 out]
                    }
                    frame 14, Default {
                    }
                  }
                }
              }
              frame #2 {
              }
            }
            n2970 = local write "OK Button 16"(FALSE ("OK Button 13")) -> ()
          }
        }
        n2971 = Index Array(array=w3690, index="Select Printer 3") -> (element=w3692:string)
        "Selected Printer" <- w3692
        n2972 = case shown="True" w3687 {
          frame False {
          }
          frame True {
            n2973 = flat-sequence {
              frame #0 {
              }
              frame #1 {
                n2974 = Wait (ms)(milliseconds to wait=u32 100) -> ()  [unwired: 1 out]
              }
              frame #2 {
                n2975 = local write "OK Button 16"(FALSE ("Print 3")) -> ()
              }
            }
          }
        }
        n2976 = case shown="True" "Print" {
          tunnel: w3692 -> [_ w3984]
          frame False {
          }
          frame True {
            (unwired) i16 6 ("width (-)")
            (unwired) "TESTED BY : "
            (unwired) "TESTED DATE :"
            (unwired) "SAMPLE ID : "
            (unwired) "SAMPLE DESIGN : "
            w3942 = "\r"
            w3959 = "\r"
            # "add image"
            n2977 = local read "Sample ID"() -> (w3932:string)
            n2978 = local read "Tested by"() -> (w3935:string)
            n2979 = local read "String 34"() -> (w3922:string)
            n2980 = local read "String 45"() -> (w3902:string)
            n2981 = local read "String 35"() -> (w3917:string)
            n2982 = local read "String 37"() -> (w3915:string)
            n2983 = local read "String 32"() -> (w3937:string)
            n2984 = local read "String 36"() -> (w3912:string)
            n2985 = local read "String 31"() -> (w3936:string)
            n2986 = local read "Test Date"() -> (w3933:string)
            n2987 = local read "String 33"() -> (w3938:string)
            n2988 = local read "String 38"() -> (w3908:string)
            n2989 = local read "String 39"() -> (w3905:string)
            n2990 = local write "Print"(FALSE ("Print FF")) -> ()
            n2991 = local read "S 39"() -> (w3920:string)
            n2992 = local read "S 38"() -> (w3927:string)
            n2993 = local read "Temperature before test 2"() -> (w3958:dbl)
            n2994 = local read "Temperature after test 2"() -> (w3948:dbl)
            n2995 = local read "Humidity before test 2"() -> (w3973:dbl)
            n2996 = local read "Humidity after test 2"() -> (w3957:dbl)
            n2997 = local read "MWSD 2"() -> (w3962:dbl)
            n2998 = local read "WS1.4 2"() -> (w3940:dbl)
            n2999 = Concatenate Strings("2)" ("string"), w3922) -> (w3923:string)
            n3000 = Concatenate Strings("3)" ("string"), w3920) -> (w3921:string)
            n3001 = Concatenate Strings("1)" ("string"), w3927) -> (w3926:string)
            n3002 = Concatenate Strings("4)" ("string"), w3917) -> (w3918:string)
            n3003 = Concatenate Strings("5)" ("string"), w3915) -> (w3914:string)
            n3004 = Concatenate Strings("6)" ("string"), w3912) -> (w3911:string)
            n3005 = Concatenate Strings("7)" ("string"), w3908) -> (w3909:string)
            n3006 = Concatenate Strings("8)" ("string"), w3905) -> (w3906:string)
            n3007 = local read "HCF 2"() -> (w3944:dbl)
            n3008 = local read "AVP 2"() -> (w3961:dbl)
            n3009 = local read "s.NO"() -> (w3903:string)
            n3010 = call <vilib>:"New Report.vi"("report type"=enum16{"Standard Report", "HTML"}."Standard Report") -> ("report out"=w3982:refnum<class "NI_report.lvclass">, "error out"=w3981:errorcluster)  [unwired: 13 in]
            n3011 = local read "TITTLE"() -> (w3934:string)
            n3012 = Concatenate Strings(w3959, w3902, w3903, w3959, w3937, w3932, w3959, w3936, w3933, w3959, w3938, w3935, w3959) -> (w3952:string)
            "test by" <- w3952
            n3013 = Number To Fractional String(number=w3958, width (-)=i16 6, precision (6)=i16 2) -> (F-format string=w3947:string)  [unwired: 1 in]
            n3014 = Number To Fractional String(number=w3957, width (-)=i16 6, precision (6)=i16 2) -> (F-format string=w3960:string)  [unwired: 1 in]
            n3015 = Number To Fractional String(number=w3973, width (-)=i16 6, precision (6)=i16 2) -> (F-format string=w3978:string)  [unwired: 1 in]
            n3016 = Number To Fractional String(number=w3962, width (-)=i16 6, precision (6)=i16 2) -> (F-format string=w3964:string)  [unwired: 1 in]
            n3017 = Number To Fractional String(number=w3948, width (-)=i16 6, precision (6)=i16 2) -> (F-format string=w3949:string)  [unwired: 1 in]
            n3018 = Number To Fractional String(number=w3961, width (-)=i16 6, precision (6)=i16 2) -> (F-format string=w3963:string)  [unwired: 1 in]
            n3019 = Number To Fractional String(number=w3944, width (-)=i16 6, precision (6)=i16 2) -> (F-format string=w3943:string)  [unwired: 1 in]
            n3020 = Number To Fractional String(number=w3940, precision (6)=i16 2) -> (F-format string=w3939:string)  [unwired: 2 in]
            n3021 = call-dynamic "Set Report Header Text.vi"("report in"=w3982, "center header text"=w3934, "error in (no error)"=w3981) -> ("report out"=w3953:refnum<class "NI_report.lvclass">, "error out"=w3954:errorcluster)  [unwired: 11 in]
            n3022 = Concatenate Strings(w3942, w3926, w3978, w3942, w3923, w3947, w3942, w3921, w3960, w3942, w3918, w3949, w3942, w3914, w3964, w3942, w3911, w3963, w3942, w3909, w3943, w3942, w3906, w3939) -> (w3930:string)
            "export 2" <- w3930
            n3023 = call-poly <vilib>:"Append Report Text.vi"("report in"=w3953, "text"=w3952, "error in (no error)"=w3954) -> ("report out"=w3956:refnum<class "NI_report.lvclass">, "error out"=w3955:errorcluster)  [unwired: 9 in, 2 out]
            n3024 = local read "test by"() -> (w3929:string)
            n3025 = local read "TITTLE"() -> (w3931:string)
            n3026 = call-poly <vilib>:"Append Report Text.vi"("report in"=w3956, "error in (no error)"=w3955) -> ("report out"=w3977:refnum<class "NI_report.lvclass">, "error out"=w3975:errorcluster)  [unwired: 10 in, 2 out]
            n3027 = Concatenate Strings(w3931, w3930, w3929) -> (→"output":string)
            n3028 = call-poly <vilib>:"Append Report Text.vi"("report in"=w3977, "text"=w3930, "error in (no error)"=w3975) -> ("report out"=w3976:refnum<class "NI_report.lvclass">, "error out"=w3974:errorcluster)  [unwired: 9 in, 2 out]
            n3029 = call-dynamic "Print Report.vi"("report in"=w3976, "printer name (default)"=w3984, "error in (no error)"=w3974) -> ("report out"=w3986:refnum<class "NI_report.lvclass">, "error out"=w3987:errorcluster)  [unwired: 11 in]
            n3030 = call-dynamic "Dispose Report.vi"("report in"=w3986, "error in (no error)"=w3987) -> ()  [unwired: 13 in, 1 out]
          }
        }
        n3031 = case shown="True" "Print 2" {
          frame False {
          }
          frame True {
            n3032 = flat-sequence {
              frame #0 {
                n3033 = local read "s.NO"() -> (→"s.NO 2":string)
                n3034 = Wait (ms)(milliseconds to wait=u32 20) -> ()  [unwired: 1 out]
                n3035 = local read "Sample ID  3"() -> (→"Sample ID  6":string)
                n3036 = local read "Sample ID  4"() -> (→"Sample ID  7":string)
                n3037 = local read "Sample ID"() -> (→"Sample ID  2":string)
                n3038 = local read "Tested by"() -> (→"Tested by 2":string)
                n3039 = local read "Test Date"() -> (→"Test Date 2":string)
                n3040 = local read "Humidity after test 3"() -> (→"Humidity after test 4":dbl)
                n3041 = local read "Ref A Test Date :"() -> (→"TITTLE 4":string)
                n3042 = local read "Temperature before test 3"() -> (w3809:dbl)
                n3043 = local read "Temperature before test 3"() -> (→"Temperature after test 5":dbl)
                n3044 = local read "Temperature after test 3"() -> (→"Temperature after test 4":dbl)
                n3045 = local read "Humidity before test 3"() -> (→"Humidity before test 4":dbl)
                n3046 = local write "Temperature before test 3"(w3809) -> ()
                n3047 = local read "image data"() -> (w3800:T16)
                n3048 = String To Path(string="C:\\LAB-IQ\\im\\Temp_resized.jpg") -> (path=w3801:path)
                "path 2" <- w3801
                n3049 = call <vilib>:"Write JPEG File.vi"("image data"=w3800, "path to JPEG file"=w3801) -> ()  [unwired: 8 in, 2 out]
                "Ref A Test Date :" <- "Ref A Test Date :"
                "Ref B Test Date :" <- "Ref B Test Date :"
                "Ref B Scar Value :" <- "Ref B Scar Value :"
                "Ref A Scar Value :" <- "Ref A Scar Value :"
              }
              frame #1 {
                (unwired) HTML_Report_Image_Alignment."MIDDLE" ("alignment (default)")
                w3837 = u16 0 items=["portrait", "landscape"] ("orientation (portrait)")
                (unwired) HTML_Report_Image_Alignment."ABSMIDDLE" ("alignment (default)")
                (unwired) "TESTED BY : "
                (unwired) "TESTED DATE :"
                (unwired) "SAMPLE ID : "
                (unwired) "SAMPLE DESIGN : "
                w3870 = "\r"
                # "add image"
                n3050 = Wait (ms)(milliseconds to wait=u32 20) -> ()  [unwired: 1 out]
                n3051 = local read "Sample ID  2"() -> (w3863:string)
                n3052 = local read "Wear Scar X"() -> (w3835:dbl)
                "Length ( microns ) 2" <- w3835
                n3053 = local read "Wear Scar Y"() -> (w3834:dbl)
                "Wear Scar Y ( microns ) :" <- w3834
                n3054 = local read "Test Date 2"() -> (w3864:string)
                n3055 = local read "Tested by 2"() -> (w3865:string)
                n3056 = local read "String 46"() -> (w3861:string)
                n3057 = local read "String 48"() -> (w3867:string)
                n3058 = local read "String 47"() -> (w3866:string)
                n3059 = local read "String 49"() -> (w3868:string)
                n3060 = local read "String 10"() -> (w3821:string)
                n3061 = local read "s.NO 2"() -> (w3862:string)
                n3062 = Add(x=w3835, y=w3834) -> (x+y=w3833:dbl)
                n3063 = call <vilib>:"New Report.vi"("report type"=enum16{"Standard Report", "HTML"}."HTML") -> ("report out"=w3841:refnum<class "NI_report.lvclass">, "error out"=w3839:errorcluster)  [unwired: 13 in]
                n3064 = Concatenate Strings(w3870, w3861, w3862, w3870, w3867, w3863, w3870, w3866, w3864, w3870, w3868, w3865, w3870) -> (→"test by 2":string)
                n3065 = Concatenate Strings("C:\\LAB-IQ\\Data\\" ("string"), w3821, ".jpg" ("string")) -> ()  [unwired: 1 out]
                n3066 = Divide(x=w3833, y=2.0) -> (x/y=→"Mean Wear ( microns) :":dbl)
                n3067 = call-dynamic "Set Report Orientation.vi"("report in"=w3841, "orientation (portrait)"=w3837, "error in (no error)"=w3839) -> ("report out"=w3840:refnum<class "NI_report.lvclass">, "error out"=w3838:errorcluster)  [unwired: 11 in]
                n3068 = for {
                  N: 5 -> [_]
                  tunnel: w3840 -> [w3891]
                  tunnel: [w3890] -> w3819
                  tunnel: w3838 -> [w3889]
                  tunnel: [w3888] -> w3818
                  n3069 = call-dynamic "Set Report Tab Width.vi"("report in"=w3891, "error in (no error)"=w3889) -> ("report out"=w3890:refnum<class "NI_report.lvclass">, "error out"=w3888:errorcluster)  [unwired: 12 in]
                }
                n3070 = local read "TITTLE"() -> (w3836:string)
                n3071 = call-dynamic "Set Report Header Text.vi"("report in"=w3819, "center header text"=w3836, "error in (no error)"=w3818) -> ("report out"=w3857:refnum<class "NI_report.lvclass">, "error out"=w3856:errorcluster)  [unwired: 11 in]
                n3072 = for {
                  N: 1 -> [_]
                  tunnel: [w3895] -> w3843
                  tunnel: [w3894] -> w3842
                  tunnel: w3857 -> [w3893]
                  tunnel: w3856 -> [w3892]
                  n3073 = call-dynamic "New Report Line.vi"("report in"=w3893, "error in (no error)"=w3892) -> ("report out"=w3895:refnum<class "NI_report.lvclass">, "error out"=w3894:errorcluster)  [unwired: 12 in]
                }
                n3074 = for {
                  N: 2 -> [_]
                  tunnel: [w3887] -> w3849
                  tunnel: [w3886] -> w3848
                  tunnel: w3843 -> [w3885]
                  tunnel: w3842 -> [w3884]
                  n3075 = call-dynamic "New Report Line.vi"("report in"=w3885, "error in (no error)"=w3884) -> ("report out"=w3887:refnum<class "NI_report.lvclass">, "error out"=w3886:errorcluster)  [unwired: 12 in]
                }
                n3076 = for {
                  N: 25 -> [_]
                  tunnel: w3849 -> [w3883]
                  tunnel: w3848 -> [w3881]
                  tunnel: [w3882] -> w3852